vi "MeasureDC120629.vi"() -> ()   [LabVIEW 2011]
uses:
  Sub VIs/Trap cluster.ctl
  <vilib>/Utility/inputDevices.llb/closeKeyboard.vi
  <vilib>/Utility/inputDevices.llb/keyboardAcquire.vi
  <vilib>/Utility/file.llb/Write To Spreadsheet File (DBL).vi
  <vilib>/vision/driver/NI_Vision_Acquisition_Software.lvlib
panel:
  in  "Generate hologram":bool
  in  "ok 2":bool caption="Mark the center of \nthe spot using the \nzoom and the point\ntool, then click this \nbutton"
  in  "Run calibration 2":bool
  in  "e_desired":sgl=0.5
  in  "View Licence":bool
  in  "Stop program":bool
  out "Camera enabled":bool
  out "SLM enabled":bool
  in  "Hologram generation":cluster{"Method":i32, "Iterations":i32}={"Method"=0, "Iterations"=10} {"Method" items=["Lenses & Gratings (3D)", " Gerchberg-Saxton (3D)", "Gerchberg-Saxton FFT (2D)"]}
  in  "Display hologram\nand computed \nimage plane":bool=TRUE
  in  "ROI":T1={"Global Rectangle"=[568, 568, 719, 569], "Contours"=[{"Contour Type"=0, "ROI Type"=1, "Points"=[568, 568]}, {"Contour Type"=0, "ROI Type"=1, "Points"=[642, 568]}, {"Contour Type"=0, "ROI Type"=1, "Points"=[718, 568]}]}
  out "Image":T2(plugin-control)
  in  "Spots x":i32
  in  "Spots y":i32
  in  "Cancel calibration 2":bool
  in  "separation step":i32=1 min=1
  in  "max separation":i32=40
  in  "min separation":i32=30
  in  "Measure":bool
  in  "#images":i32=1
  out "Step number":i32
  in  "Move one spot":bool
  in  "y":dbl=100.0 min=1e-22
  in  "Filename":string="test"
  out "appended path":path=path "C:/Users/Martin/Dropbox/GU/CUDA/GenerateHologramCUDA/LabVIEW/MartinDC/Measurements/test0_0.bmp"
  in  "File Path":path=path "C:/Users/Martin/Dropbox/GU/CUDA/GenerateHologramCUDA/LabVIEW/MartinDC/Measurements"
  in  "Show image":bool=TRUE
  in  "ROI size":dbl=2.0 min=2.0 step=2.0
  out "Calculated image plane":dbl[][](graph)
  out "Current trap pos":T3={"X (IMAQ)"=[555.0, 642.5, 730.0, 555.0, 642.5, 730.0, 555.0, 642.5, 730.0], "Y (IMAQ)"=[555.0, 555.0, 555.0, 642.5, 642.5, 642.5, 730.0, 730.0, 730.0], "Z"=[0.0, 0.0, 0.0, 0.0, 0.0, 0.0, 0.0, 0.0, 0.0], "Amplitudes"=[1.0, 1.0, 1.0, 1.0, 1.0, 1.0, 1.0, 1.0, 1.0], "Trap number"=[0, 1, 2, 3, 4, 5, 6, 7, 8], "ROI number"=[0, 1, 2, 3, 4, 5, 6, 7, 8], "Number of traps"=9, "Group"=[FALSE, FALSE, FALSE, FALSE, FALSE, FALSE, FALSE, FALSE, FALSE]}
  out "NI Vision error":errorcluster
  out "CUDA/SLM error":errorcluster
  in  "Display path":bool=TRUE
  out "Displayed Hologram":u8[][](graph)
  in  "Coordinate mapping \n(IMAQ to SLM)":T4={"sX"=-256.0, "sY"=-256.0, "sZ"=0.0, "cX"=0.4, "cY"=0.4, "cZ"=1.0}
  in  "Switch X/Y":bool
  # "Martin\nPersson 2011"
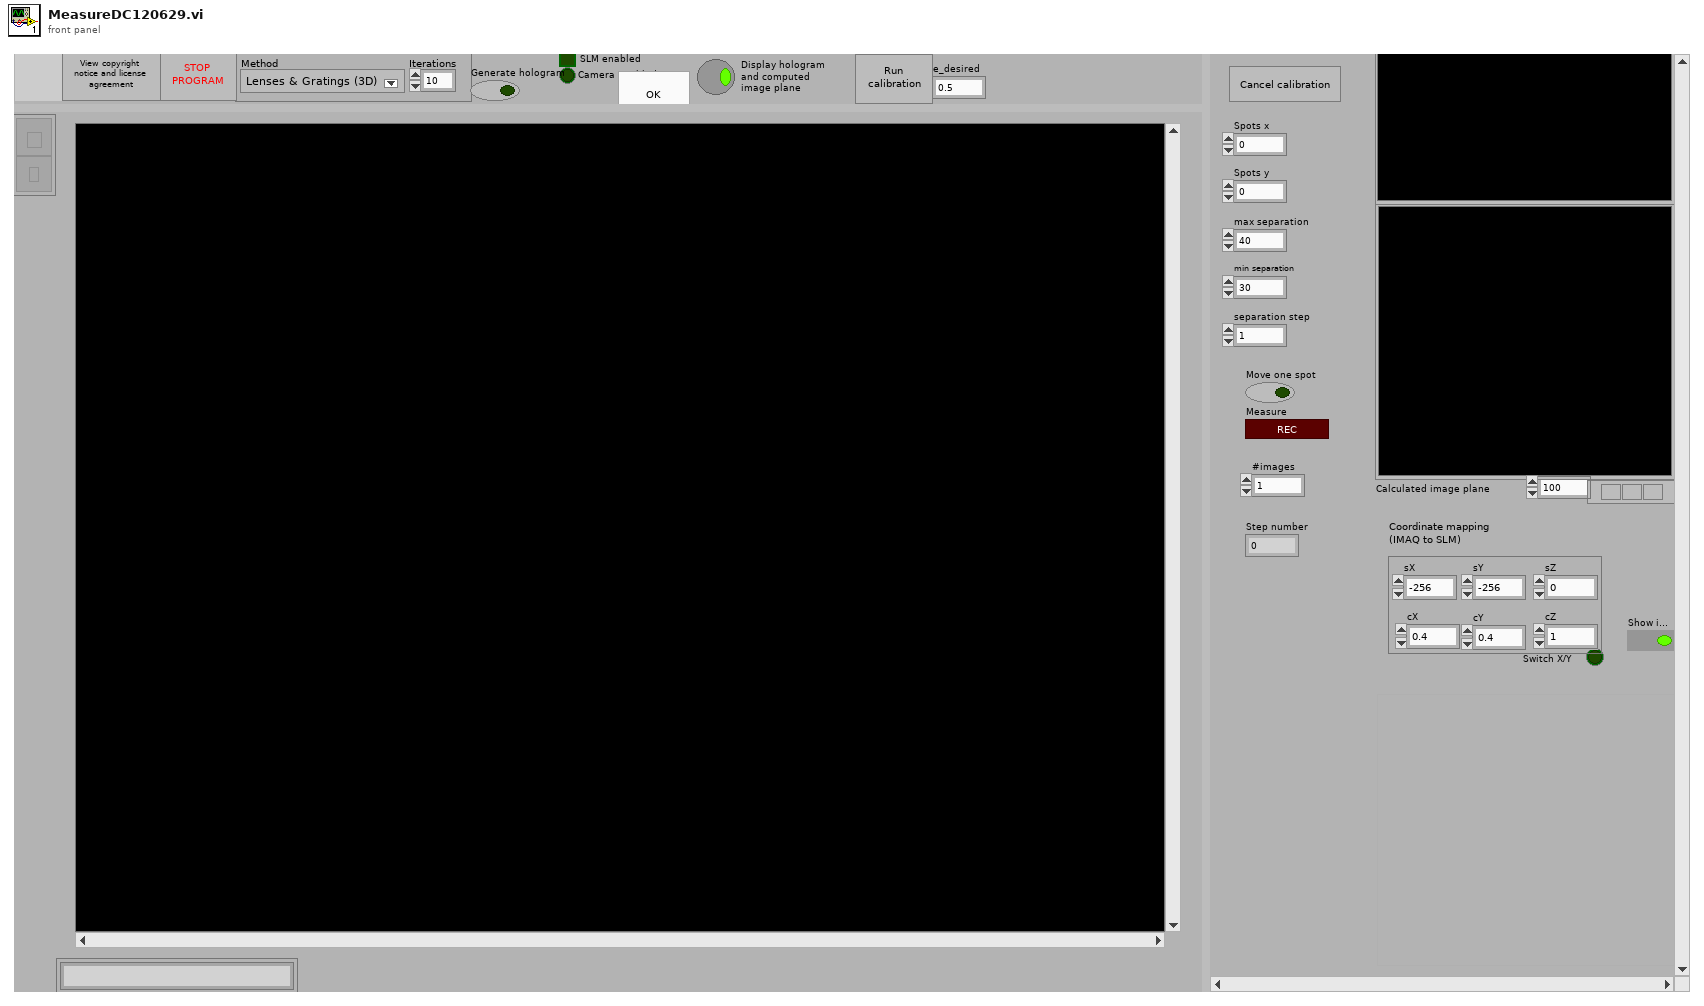
[diagram p1: front panel]
types:
  T1 = cluster{"Global Rectangle":i32[], "Contours":cluster{"Contour Type":u32, "ROI Type":u32, "Points":i32[]}[]}
  T2 = typedef "IMAQ Image.ctl" = refnum<image>
  T3 = typedef "Trap cluster.ctl" = cluster{"X (IMAQ)":dbl[], "Y (IMAQ)":dbl[], "Z":dbl[], "Amplitudes":dbl[], "Trap number":i32[], "ROI number":i32[], "Number of traps":i32, "Group":bool[]}
  T4 = cluster{"sX":dbl, "sY":dbl, "sZ":dbl, "cX":dbl, "cY":dbl, "cZ":dbl}
  T5 = cluster{"Centroid X":dbl[], "Centroid Y":dbl[], "Acquired Buffer Number":u32}
  T6 = typedef "IMAQdx.ctl" = refnum<k21>
  T7 = enum16{"0", "1", "2", "3", "4", "5", "6", "7", "8", "9", "A", "B", "C", "D", "E", "F", "G", "H", "I", "J", "K", "L", "M", "N", "O", "P", "Q", "R", "S", "T", "U", "V", "W", "X", "Y", "Z", "F1", "F2", "F3", "F4", "F5", "F6", "F7", "F8", "F9", "F10", "F11", "F12", "F13", "F14", "F15", "ADD", "BACK", "BACKSLASH", "CAPITAL", "COMMA", "DECIMAL", "DELETE", "DIVIDE", "DOWN", "END", "EQUALS", "ESCAPE", "GRAVE (`)", "HOME", "INSERT", "LBRACKET", "LCONTROL", "LEFT", "L ALT", "LSHIFT", "LWIN", "MINUS", "MULTIPLY", "NEXT", "NUMLOCK", "NUMPAD_0", "NUMPAD_1", "NUMPAD_2", "NUMPAD_3", "NUMPAD_4", "NUMPAD_5", "NUMPAD_6", "NUMPAD_7", "NUMPAD_8", "NUMPAD_9", "PAUSE", "PERIOD", "PRIOR (PG UP)", "RBRACKET", "RCONTROL", "RETURN", "RIGHT", "R ALT", "RSHIFT", "RWIN", "SCROLL", "SEMICOLON", "SLASH", "SPACE", "SUBTRACT", "TAB", "UP", "ENTER (num pad)", "' (quote)"}[]
  T8 = typedef "LVRectTypeDef.ctl" = cluster{"left":i16, "top":i16, "right":i16, "bottom":i16}
  T9 = cluster{"Contour Type":u32, "ROI Type":u32, "Points":i32[]}[]
  T10 = cluster{"Contour Type":u32, "ROI Type":u32, "Points":i32[]}
  T11 = typedef "Semaphore RefNum" = refnum<k1>
  T12 = typedef "Image Type" = u32
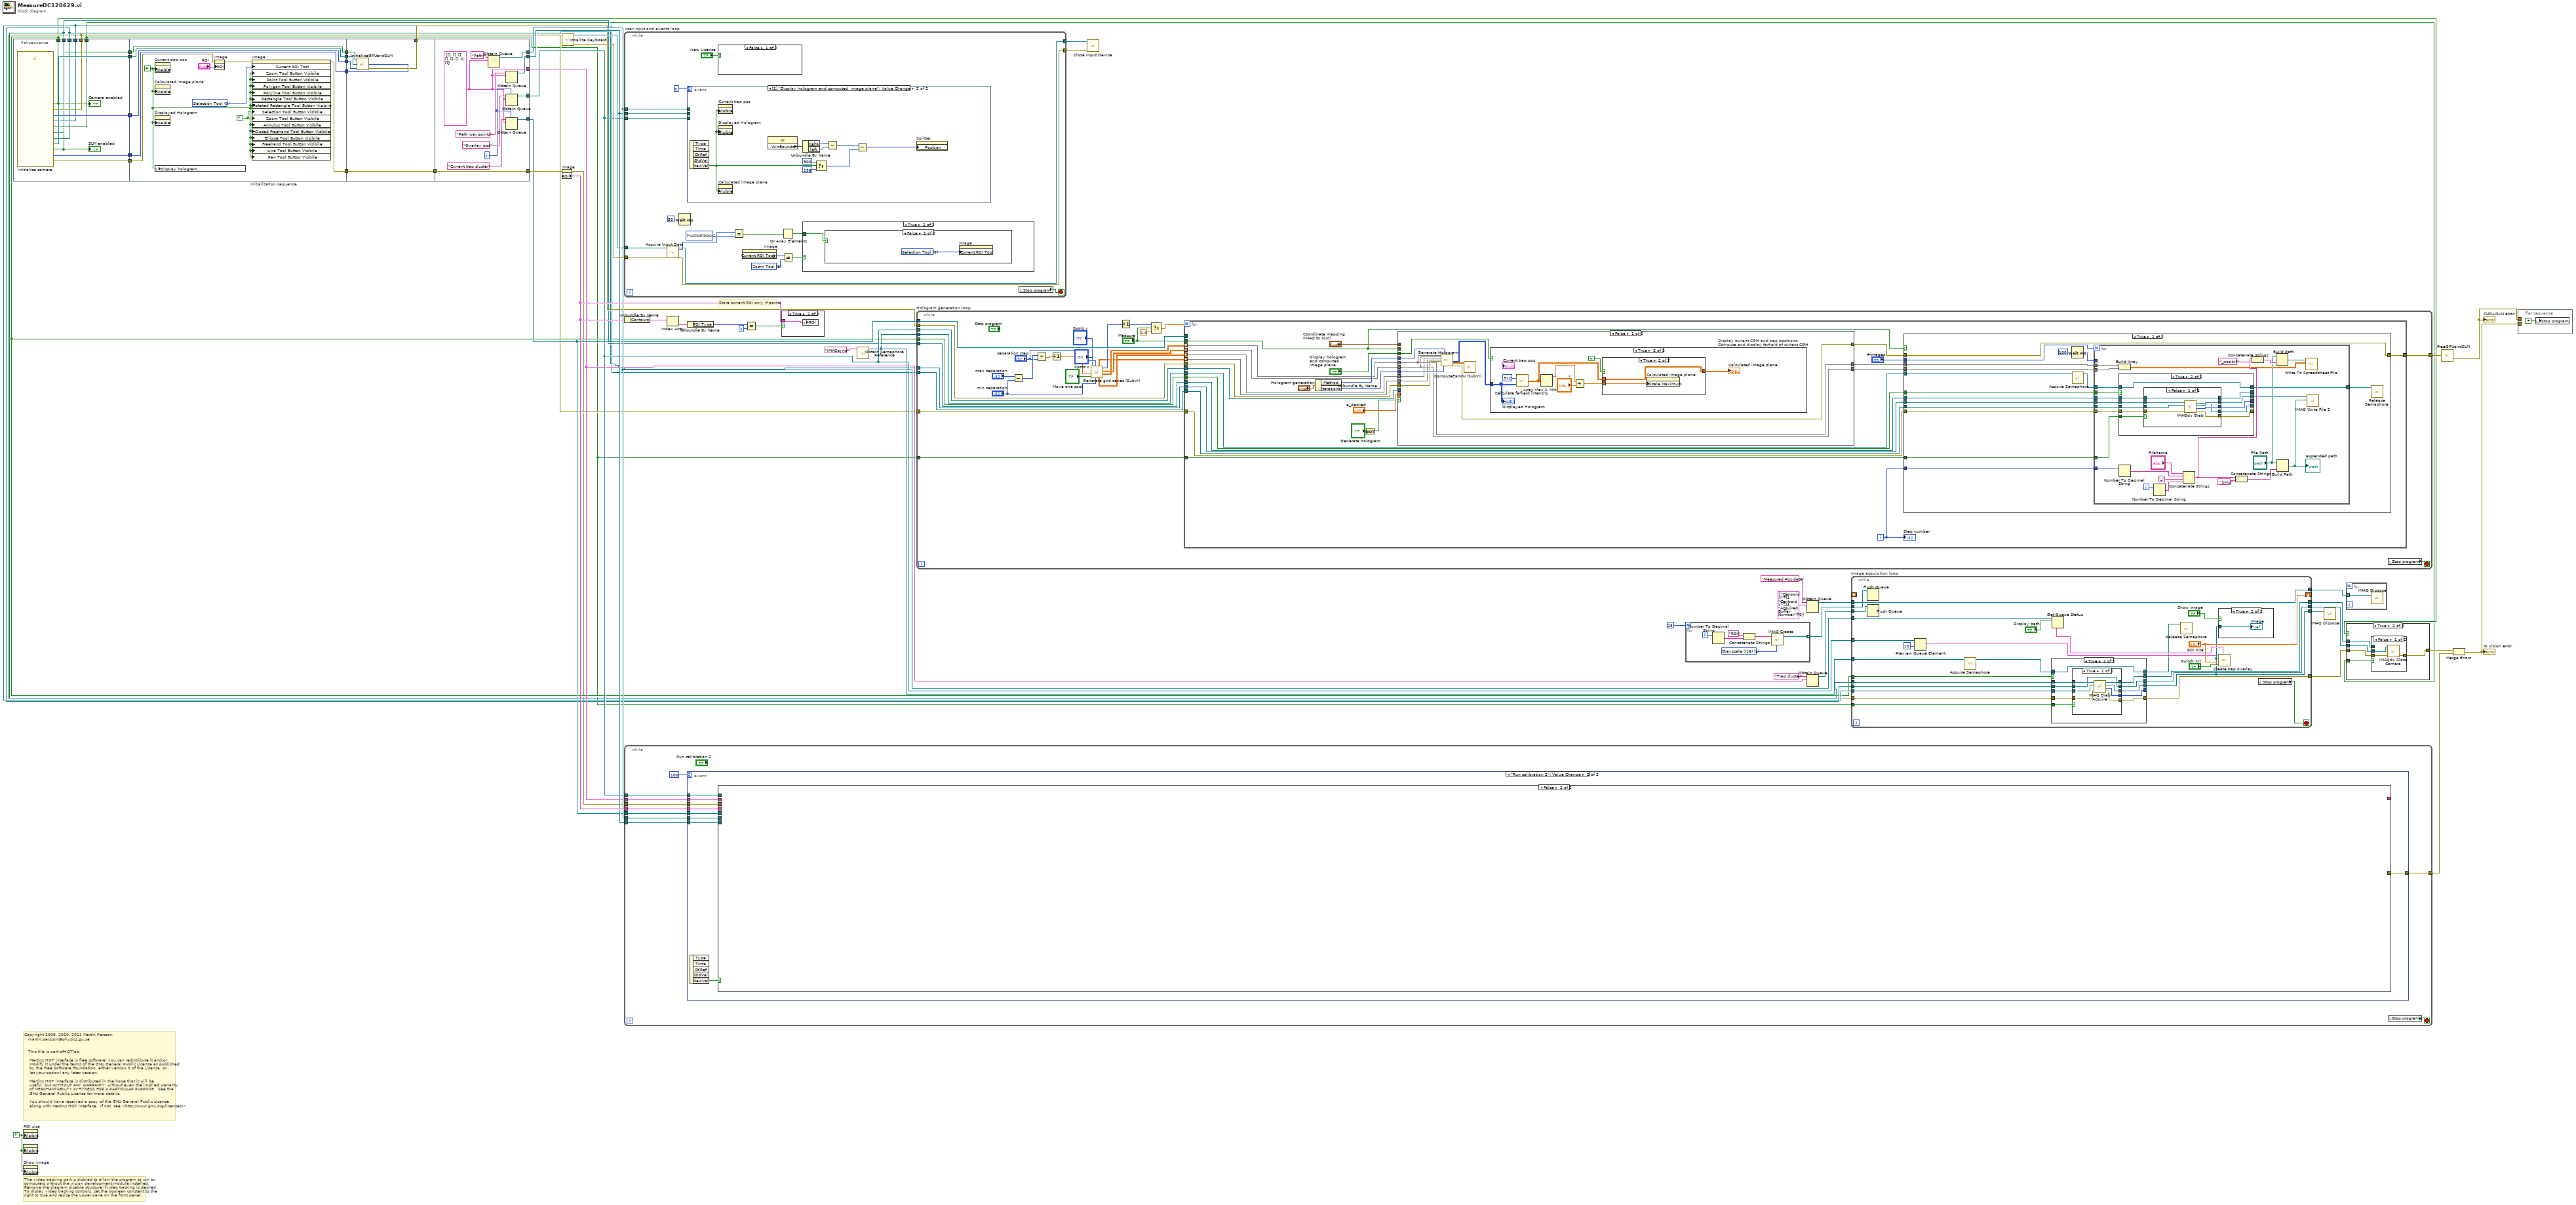
[diagram p0: block diagram]
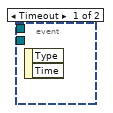
[diagram p2: hidden frame]
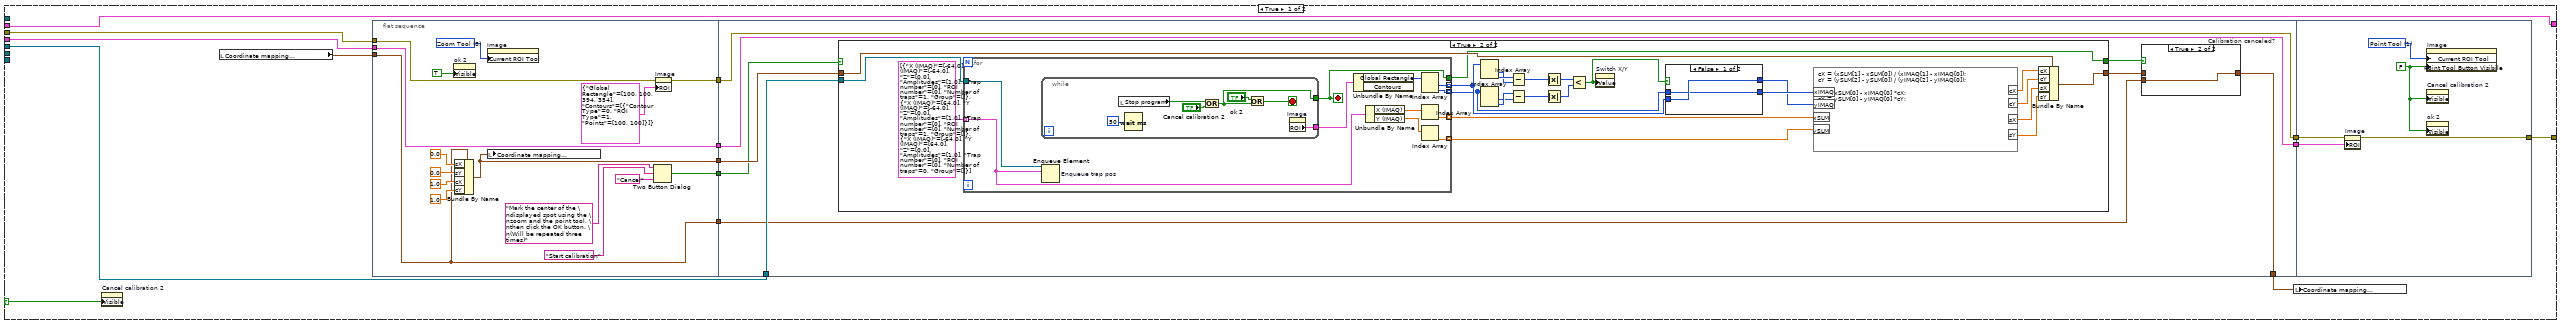
[diagram p3: hidden frame]
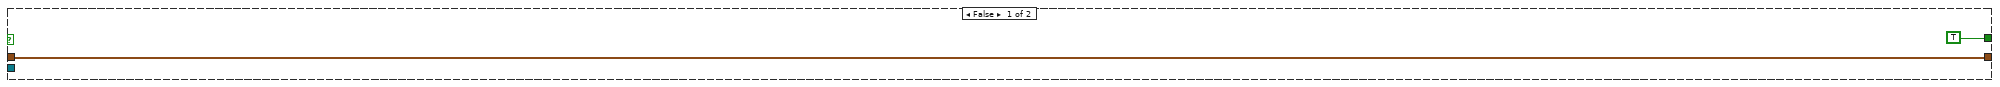
[diagram p5: hidden frame]
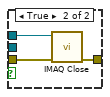
[diagram p8: hidden frame]
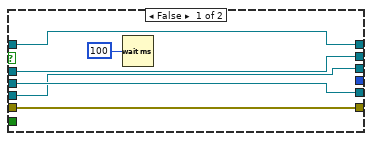
[diagram p10: hidden frame]
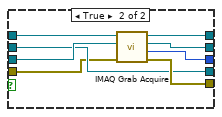
[diagram p11: hidden frame]
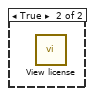
[diagram p15: hidden frame]
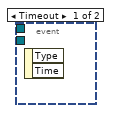
[diagram p16: hidden frame]
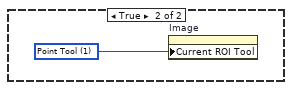
[diagram p18: hidden frame]
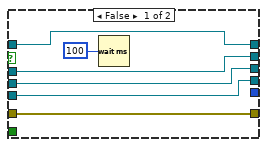
[diagram p20: hidden frame]
diagram:
  w42 = TRUE ("Visible")
  # "Copyright 2009, 2010, 2011 Martin Persson \n   martin.persson@physics.gu.se\n\n\n   This file is part ofHOTlab.\n\n    Martins HOT interface is free software: you can redistribute it and/or \n    modify it under the terms of the GNU General Public License as published \n    by the Free Software Foundation, either version 3 of the License, or\n    (at your option) any later version.\n\n    Martins HOT interface is distributed in the hope that it will be \n    useful, but WITHOUT ANY WARRANTY; without even the implied warranty\n    of MERCHANTABILITY or FITNESS FOR A PARTICULAR PURPOSE.  See the\n    GNU General Public License for more details.\n\n    You should have received a copy of the GNU General Public License\n    along with Martins HOT interface.  If not, see <http://www.gnu.org/licenses/>."
  # "Store current ROI only if points"
  # "The video tracking part is disbled to allow the program to run on\ncomputers without the vision development module installed. \nRemove the diagram disable structure ifvideo tracking is desired. \nTo diplay video tracking controls, set the boolean constant to the \nright to true And resize the upper pane on the front panel."
  n1 = flat-sequence "Initialization sequence" {
    tunnel: [w57] -> w27
    tunnel: [w66] -> w26
    tunnel: [w65] -> w25
    tunnel: [w64] -> w24
    tunnel: [w63] -> w23
    tunnel: [w62] -> w7
    tunnel: [w61] -> w8
    tunnel: [w60] -> w6
    tunnel: [w59] -> w4
    tunnel: [w58] -> w9
    tunnel: [w56] -> w5
    tunnel: w27 -> [w74]
    tunnel: w26 -> [w72]
    tunnel: w25 -> [w77]
    tunnel: w24 -> [w76]
    tunnel: w23 -> [w75]
    tunnel: [w74] -> w16
    tunnel: [w67] -> w15
    tunnel: [w77] -> w13
    tunnel: [w76] -> w12
    tunnel: [w75] -> w11
    tunnel: w16 -> [w80]
    tunnel: w15 -> [w83]
    tunnel: [w83] -> w14
    tunnel: w13 -> [w81]
    tunnel: w12 -> [w82]
    tunnel: w11 -> [w79]
    tunnel: [w78] -> w10
    tunnel: [w94] -> w22
    tunnel: w14 -> [w94]
    tunnel: [w92] -> w21
    tunnel: [w90] -> w20
    tunnel: [w88] -> w19
    tunnel: [w87] -> w18
    tunnel: [w84] -> w17
    frame #0 {
      n2 = call "Initialize camera.vi"() -> ("CUDA device ID"=w64:i32, "IMAQdx Session Out"=w61:T6, "TrueFrame out"=w65:i32, "IMAQ camera"=w59:bool, "Image reference out"=w62:T2, "SLM enabled"=w57:bool, "Camera enabled"=w56:bool, "Vision error out"=w66:errorcluster, "LUT path out"=w63:path, "IMAQ Session Out"=w58:refnum<k11>, "Camera error"=w60:errorcluster)  [unwired: 5 in]
      "Camera enabled" <- w56
      "SLM enabled" <- w57
    }
    frame #1 {
      w70 = TRUE ("ROI Tool Buttons Visibile:Zoom Tool Button Visible")
      w71 = FALSE ("ROI Tool Buttons Visibile:Zoom Tool Button Visible")
      w69 = u32 0 items=["Zoom Tool"=8, "Selection Tool"=0, "Pan Tool"=9, "Point Tool"=1, "Line Tool"=2, "Rectangle Tool"=3, "Rotated Rectangle Tool"=12, "Polyline Tool"=10, "Polygon Tool"=5, "Freehand Tool"=11, "Closed Freehand Tool"=6, "Ellipse Tool"=4, "Annulus Tool"=7] ("Current ROI Tool")
      n3 = property on="Current trap pos" class="Clust (strict)"("Visible"=w71) -> ()  [unwired: 2 in, 2 out]
      n4 = property on="Calculated image plane" class="IntGraph (strict)"("Visible"=w71) -> ()  [unwired: 2 in, 2 out]
      n5 = property on="Displayed Hologram" class="IntGraph (strict)"("Visible"=w71) -> ()  [unwired: 2 in, 2 out]
      n6 = local write "Display hologram\nand computed \nimage plane"(w71) -> ()
      n7 = property on="Image" class="ImageControl"(error in=w72, "ROI"="ROI") -> (error out=w68:errorcluster)  [unwired: 1 in, 1 out]
      n8 = property on="Image" class="ImageControl"(error in=w68, "Current ROI Tool"=w69, "Zoom Tool Button Visibile"=w71, "Point Tool Button Visibile"=w71, "Polygon Tool Button Visibile"=w71, "Polyline Tool Button Visibile"=w71, "Rectangle Tool Button Visibile"=w71, "Rotated Rectangle Tool Button Visibile"=w71, "Selection Tool Button Visibile"=w70, "Zoom Tool Button Visibile"=w70, "Annulus Tool Button Visibile"=w71, "Closed Freehand Tool Button Visibile"=w71, "Ellipse Tool Button Visibile"=w71, "Freehand Tool Button Visibile"=w71, "Line Tool Button Visibile"=w71, "Pan Tool Button Visibile"=w71) -> (error out=w67:errorcluster)  [unwired: 1 in, 1 out]
    }
    frame #2 {
      n9 = call "InitializeGPUandSLM.vi"("TrueFrame"=w81, "deviceId"=w82, "Path to LUT file"=w79, "SLM enabled"=w80) -> ("CUDA/SLM error"=w78:errorcluster)  [unwired: 1 out]
    }
    frame #3 {
      w85 = 1 ("max queue size (-1, unlimited)")
      w84 = T3 {"X (IMAQ)"=[], "Y (IMAQ)"=[], "Z"=[], "Amplitudes"=[], "Trap number"=[], "ROI number"=[], "Number of traps"=0, "Group"=[]} ("output cluster 2")
      n10 = Obtain Queue(name (unnamed)="Path", element data type=w84) -> (queue out=w92:refnum<queue>)  [unwired: 3 in, 2 out]
      n11 = Obtain Queue(name (unnamed)="Path waypoints", element data type=w84) -> (queue out=w90:refnum<queue>)  [unwired: 3 in, 2 out]
      n12 = Obtain Queue(max queue size (-1, unlimited)=w85, name (unnamed)="Overlay pos", element data type=w84) -> (queue out=w87:refnum<queue>)  [unwired: 2 in, 2 out]
      n13 = Obtain Queue(max queue size (-1, unlimited)=w85, name (unnamed)="Current trap cluster", element data type=w84) -> (queue out=w88:refnum<queue>)  [unwired: 2 in, 2 out]
    }
  }
  n14 = property on="ROI size" class="DigNum (strict)"("Visible"=w42) -> ()  [unwired: 2 in, 2 out]
  n15 = property on="Measure" class="Bool"("Visible"=w42) -> ()  [unwired: 2 in, 2 out]
  n16 = property on="Show image" class="Bool (strict)"("Visible"=w42) -> ()  [unwired: 2 in, 2 out]
  n17 = call <vilib>:"Intialize Keyboard.vi"() -> ("error out"=w29:errorcluster, "device ID"=w55:refnum<k1>)  [unwired: 1 in, 9 out]
  n18 = property on="Image" class="ImageControl"(error in=w22) -> (error out=w1:errorcluster, "ROI"=w36:T1)  [unwired: 1 in, 1 out]
  n19 = while "User input and events loop" {
    tunnel: w55 -> [w112]
    tunnel: w18 -> [w101]
    tunnel: w20 -> [w100]
    tunnel: w21 -> [w99]
    tunnel: [w98] -> w30
    tunnel: w29 -> [w97]
    tunnel: [w96] -> w28
    stop <- w104 stop-if-true
    w109 = u32 8 items=["Zoom Tool"=8, "Selection Tool"=0, "Pan Tool"=9, "Point Tool"=1, "Line Tool"=2, "Rectangle Tool"=3, "Rotated Rectangle Tool"=12, "Polyline Tool"=10, "Polygon Tool"=5, "Freehand Tool"=11, "Closed Freehand Tool"=6, "Ellipse Tool"=4, "Annulus Tool"=7] ("Current ROI Tool")
    w106 = T7 [enum."LCONTROL"] items=["0", "1", "2", "3", "4", "5", "6", "7", "8", "9", "A", "B", "C", "D", "E", "F", "G", "H", "I", "J", "K", "L", "M", "N", "O", "P", "Q", "R", "S", "T", "U", "V", "W", "X", "Y", "Z", "F1", "F2", "F3", "F4", "F5", "F6", "F7", "F8", "F9", "F10", "F11", "F12", "F13", "F14", "F15", "ADD", "BACK", "BACKSLASH", "CAPITAL", "COMMA", "DECIMAL", "DELETE", "DIVIDE", "DOWN", "END", "EQUALS", "ESCAPE", "GRAVE (`)", "HOME", "INSERT", "LBRACKET", "LCONTROL", "LEFT", "L ALT", "LSHIFT", "LWIN", "MINUS", "MULTIPLY", "NEXT", "NUMLOCK", "NUMPAD_0", "NUMPAD_1", "NUMPAD_2", "NUMPAD_3", "NUMPAD_4", "NUMPAD_5", "NUMPAD_6", "NUMPAD_7", "NUMPAD_8", "NUMPAD_9", "PAUSE", "PERIOD", "PRIOR (PG UP)", "RBRACKET", "RCONTROL", "RETURN", "RIGHT", "R ALT", "RSHIFT", "RWIN", "SCROLL", "SEMICOLON", "SLASH", "SPACE", "SUBTRACT", "TAB", "UP", "ENTER (num pad)", "' (quote)"] ("keys pressed")
    n20 = call-poly <vilib>:"Acquire Input Data.vi"("device ID"=w112, "error in (no error)"=w97) -> ("device ID"=w98:refnum<k1>, "keys pressed"=w105:T7, "error out"=w96:errorcluster)  [unwired: 15 out]
    n21 = Wait (ms)(milliseconds to wait=u32 50) -> ()  [unwired: 1 out]
    n22 = event shown="[1] \"Display hologram\nand computed \nimage plane\": Value Change" {
      selector: _ -> [_ _]
      dyn-events: _ -> [_ _]
      timeout: 0 -> [_ _]
      tunnel: w101 -> [_ _]
      tunnel: w100 -> [_ _]
      tunnel: w99 -> [_ _]
      event Timeout {
        n23 = event-data() -> ()  [unwired: 1 in, 2 out]
      }
      event "Display hologram\nand computed \nimage plane": Value Change {
        n24 = event-data() -> ("NewVal"=w114:bool)  [unwired: 1 in, 4 out]
        n25 = property on="Current trap pos" class="Clust (strict)"("Visible"=w114) -> ()  [unwired: 2 in, 2 out]
        n26 = property on="Displayed Hologram" class="IntGraph (strict)"("Visible"=w114) -> ()  [unwired: 2 in, 2 out]
        n27 = property on="Calculated image plane" class="IntGraph (strict)"("Visible"=w114) -> ()  [unwired: 2 in, 2 out]
        n28 = property on="Property Node" class="VI"() -> ("Front Panel.WinBounds"=w121:T8)  [unwired: 2 in, 2 out]
        n29 = Unbundle By Name(w121) -> ("right"=w120:i16, "left"=w119:i16)
        n30 = Select(t=i16 500 ("x-y"), s=w114, f=i16 196 ("x-y")) -> (s? t:f=w113:i16)
        n31 = Subtract(x=w120, y=w119) -> (x-y=w118:i16)
        n32 = Subtract(x=w118, y=w113) -> (x-y=w117:i16)
        n33 = property on="Splitter" class="Splitter"("Position"=w117) -> ()  [unwired: 2 in, 2 out]
      }
    }
    n34 = case shown="False" "View Licence" {
      frame False {
      }
      frame True {
        n35 = call "View license.vi"() -> ()  [unwired: 1 in]
      }
    }
    n36 = Equal?(x=w105, y=w106) -> (x = y?=w107:bool[])
    n37 = property on="Image" class="ImageControl"() -> ("Current ROI Tool"=w108:u32)  [unwired: 2 in, 2 out]
    n38 = Or Array Elements(Boolean array=w107) -> (logical OR=w111:bool)
    n39 = Not Equal?(x=w108, y=w109) -> (x != y?=w110:bool)
    n40 = case shown="True" w110 {
      tunnel: w111 -> [_ w122]
      frame False {
      }
      frame True {
        n41 = case shown="False" w122 {
          frame False {
            w123 = u32 0 items=["Zoom Tool"=8, "Selection Tool"=0, "Pan Tool"=9, "Point Tool"=1, "Line Tool"=2, "Rectangle Tool"=3, "Rotated Rectangle Tool"=12, "Polyline Tool"=10, "Polygon Tool"=5, "Freehand Tool"=11, "Closed Freehand Tool"=6, "Ellipse Tool"=4, "Annulus Tool"=7] ("Current ROI Tool")
            n42 = property on="Image" class="ImageControl"("Current ROI Tool"=w123) -> ()  [unwired: 2 in, 2 out]
          }
          frame True {
            w124 = u32 1 items=["Zoom Tool"=8, "Selection Tool"=0, "Pan Tool"=9, "Point Tool"=1, "Line Tool"=2, "Rectangle Tool"=3, "Rotated Rectangle Tool"=12, "Polyline Tool"=10, "Polygon Tool"=5, "Freehand Tool"=11, "Closed Freehand Tool"=6, "Ellipse Tool"=4, "Annulus Tool"=7] ("Current ROI Tool")
            n43 = property on="Image" class="ImageControl"("Current ROI Tool"=w124) -> ()  [unwired: 2 in, 2 out]
          }
        }
      }
    }
    n44 = local read "Stop program"() -> (w104:bool)
  }
  n45 = Unbundle By Name(w36) -> ("Contours"=w41:T9)
  n46 = while {
    tunnel: w36 -> [w134]
    tunnel: [w133] -> w34
    tunnel: w21 -> [w132]
    tunnel: w20 -> [w131]
    tunnel: w19 -> [w130]
    tunnel: w18 -> [w129]
    tunnel: w17 -> [w128]
    tunnel: w1 -> [w127]
    stop <- w125 stop-if-true
    n47 = event shown="[1] \"Run calibration 2\": Value Change" {
      selector: _ -> [_ _]
      dyn-events: _ -> [_ _]
      timeout: 100 -> [_ _]
      tunnel: w134 -> [_ w143]
      tunnel: [_ w142] -> w133
      tunnel: w132 -> [_ w141]
      tunnel: w131 -> [_ w140]
      tunnel: w130 -> [_ w139]
      tunnel: w129 -> [_ w138]
      tunnel: w128 -> [_ w137]
      tunnel: w127 -> [_ w136]
      event Timeout {
        n48 = event-data() -> ()  [unwired: 1 in, 2 out]
      }
      event "Run calibration 2": Value Change {
        n49 = event-data() -> ("NewVal"=w135:bool)  [unwired: 1 in, 4 out]
        n50 = case shown="False" w135 {
          selector: w135 -> [w145 _]
          tunnel: w140 -> [_ _]
          tunnel: w137 -> [w144 _]
          tunnel: [w144 _] -> _
          tunnel: w139 -> [w154 _]
          tunnel: w141 -> [_ _]
          tunnel: w138 -> [_ _]
          tunnel: w143 -> [w153 _]
          tunnel: w136 -> [w149 _]
          tunnel: [w146 _] -> w142
          frame True {
            n51 = property on="Cancel calibration 2" class="Bool"("Visible"=w145) -> ()  [unwired: 2 in, 2 out]
            n52 = local read "Coordinate mapping \n(IMAQ to SLM)"() -> (w152:T4)
            n53 = flat-sequence {
              tunnel: [w168] -> w158
              tunnel: [w170] -> w157
              tunnel: w153 -> [w168]
              tunnel: w152 -> [w162]
              tunnel: [w159] -> w151
              tunnel: [w162] -> w150
              tunnel: w149 -> [w161]
              tunnel: [w160] -> w147
              tunnel: [w183] -> w156
              tunnel: w158 -> [w183]
              tunnel: w157 -> [w177]
              tunnel: [w179] -> w155
              tunnel: w154 -> [w182]
              tunnel: w151 -> [w181]
              tunnel: w150 -> [w178]
              tunnel: [w175] -> w148
              tunnel: w147 -> [w175]
              tunnel: w156 -> [w238]
              tunnel: w148 -> [w236]
              tunnel: [w235] -> w146
              frame #0 {
                w171 = u32 8 items=["Zoom Tool"=8, "Selection Tool"=0, "Pan Tool"=9, "Point Tool"=1, "Line Tool"=2, "Rectangle Tool"=3, "Rotated Rectangle Tool"=12, "Polyline Tool"=10, "Polygon Tool"=5, "Freehand Tool"=11, "Closed Freehand Tool"=6, "Ellipse Tool"=4, "Annulus Tool"=7] ("Current ROI Tool")
                n54 = property on="ok 2" class="Bool"("Visible"=TRUE ("ROI Tool Buttons Visibile:Zoom Tool Button Visible")) -> ()  [unwired: 2 in, 2 out]
                n55 = Bundle By Name(cluster=w162, "sX"=0.0, "sY"=0.0, "cX"=1.0 ("sX"), "cY"=1.0) -> (w159:T4)
                n56 = property on="Image" class="ImageControl"("Current ROI Tool"=w171) -> ()  [unwired: 2 in, 2 out]
                n57 = local write "Coordinate mapping \n(IMAQ to SLM)"(w159) -> ()
                n58 = Two Button Dialog(message="Mark the center of the \ndisplayed spot using the \nzoom and the point tool, \nthen click the OK button. \n(Will be repeated three times)", 1:"Cancel" ("F button name (\"Cancel\")"), 2:"Start calibration" ("T button name (\"OK\")")) -> (T button?=w170:bool)
                n59 = property on="Image" class="ImageControl"(error in=w161, "ROI"=T1 {"Global Rectangle"=[100, 100, 394, 354], "Contours"=[{"Contour Type"=0, "ROI Type"=1, "Points"=[100, 100]}]} ("ROI 2")) -> (error out=w160:errorcluster)  [unwired: 1 in, 1 out]
              }
              frame #1 {
                n60 = case shown="True" w177 {
                  tunnel: w181 -> [w187 w198]
                  tunnel: [w187 w193] -> w180
                  tunnel: w182 -> [_ w189]
                  tunnel: [TRUE ("Stop program") w188] -> w176
                  frame False {
                  }
                  frame True {
                    n61 = for {
                      tunnel: [w225] -> w207 mode=indexing
                      tunnel: [w224] -> w206 mode=indexing
                      tunnel: T3[] [{"X (IMAQ)"=[-64.0], "Y (IMAQ)"=[-64.0], "Z"=[0.0], "Amplitudes"=[1.0], "Trap number"=[0], "ROI number"=[0], "Number of traps"=1, "Group"=[]}, {"X (IMAQ)"=[64.0], "Y (IMAQ)"=[-64.0], "Z"=[0.0], "Amplitudes"=[1.0], "Trap number"=[0], "ROI number"=[0], "Number of traps"=1, "Group"=[]}, {"X (IMAQ)"=[-64.0], "Y (IMAQ)"=[64.0], "Z"=[0.0], "Amplitudes"=[1.0], "Trap number"=[0], "ROI number"=[0], "Number of traps"=0, "Group"=[]}] -> [w222] mode=indexing
                      tunnel: [w219] -> w191 mode=indexing
                      tunnel: [w217] -> w190 mode=indexing
                      tunnel: w189 -> [w221]
                      tunnel: [w216] -> w188
                      stop <- w216 stop-if-true
                      n62 = while {
                        tunnel: [w232] -> w223
                        tunnel: [w228] -> w216
                        stop <- w230 stop-if-true
                        n63 = local read "Stop program"() -> (w229:bool)
                        n64 = Wait (ms)(milliseconds to wait=u32 50) -> ()  [unwired: 1 out]
                        n65 = Or(x=w229, y="Cancel calibration 2") -> (x .or. y?=w228:bool)
                        n66 = Or(x="ok 2", y=w228) -> (x .or. y?=w230:bool)
                        n67 = property on="Image" class="ImageControl"() -> ("ROI"=w232:T1)  [unwired: 2 in, 2 out]
                      }
                      n68 = Enqueue Element "Enqueue trap pos"(queue=w221, element=w222) -> ()  [unwired: 2 in, 3 out]
                      n69 = Unbundle By Name(w223) -> ("Global Rectangle"=w226:i32[])  [unwired: 1 out]
                      n70 = Unbundle By Name(w222) -> ("X (IMAQ)"=w220:dbl[], "Y (IMAQ)"=w218:dbl[])
                      n71 = Index Array(array=w226) -> (element #1=w225:i32, element #2=w224:i32)  [unwired: 2 in]
                      n72 = Index Array(array=w220) -> (element=w219:dbl)  [unwired: 1 in]
                      n73 = Index Array(array=w218) -> (element=w217:dbl)  [unwired: 1 in]
                    }
                    n74 = Index Array(array=w207) -> (element #1=w210:i32, element #2=w211:i32)  [unwired: 2 in]
                    n75 = Index Array(array=w206) -> (element #1=w208:i32, element #2=w209:i32)  [unwired: 2 in]
                    n76 = Subtract(x=w211, y=w210) -> (x-y=w203:i32)
                    n77 = Subtract(x=w209, y=w208) -> (x-y=w201:i32)
                    n78 = Absolute Value(x=w203) -> (abs(x)=w202:i32)
                    n79 = Absolute Value(x=w201) -> (abs(x)=w200:i32)
                    n80 = Less?(x=w202, y=w200) -> (x < y?=w199:bool)
                    n81 = property on="Switch X/Y" class="Bool (strict)"("Value"=w199) -> ()  [unwired: 2 in, 2 out]
                    n82 = case shown="False" w199 {
                      tunnel: w207 -> [w213 w215]
                      tunnel: w206 -> [w212 w214]
                      tunnel: [w212 w215] -> w204
                      tunnel: [w213 w214] -> w205
                      frame False {
                      }
                      frame True {
                      }
                    }
                    n83 = formula code="cX = (xSLM[1] - xSLM[0]) / (xIMAQ[1] - xIMAQ[0]); \ncY = (ySLM[2] - ySLM[0]) / (yIMAQ[2] - yIMAQ[0]); \n\nsX = xSLM[0] - xIMAQ[0] *cX;\nsY = ySLM[0] - yIMAQ[0] *cY;"("xIMAQ"=w205, "yIMAQ"=w204, "xSLM"=w191, "ySLM"=w190) -> ("cX"=w197:dbl, "cY"=w196:dbl, "sX"=w195:dbl, "sY"=w194:dbl)
                    n84 = Bundle By Name(cluster=w198, "cX"=w197, "cY"=w196, "sX"=w195, "sY"=w194) -> (w193:T4)
                  }
                }
                n85 = case "Calibration canceled?" shown="True" w176 {
                  tunnel: w180 -> [w184 _]
                  tunnel: [w184 w185] -> w179
                  tunnel: w178 -> [_ w185]
                  frame False {
                  }
                  frame True {
                  }
                }
              }
              frame #2 {
                w234 = FALSE ("ROI Tool Buttons Visibile:Zoom Tool Button Visible")
                w237 = u32 1 items=["Zoom Tool"=8, "Selection Tool"=0, "Pan Tool"=9, "Point Tool"=1, "Line Tool"=2, "Rectangle Tool"=3, "Rotated Rectangle Tool"=12, "Polyline Tool"=10, "Polygon Tool"=5, "Freehand Tool"=11, "Closed Freehand Tool"=6, "Ellipse Tool"=4, "Annulus Tool"=7] ("Current ROI Tool")
                n86 = property on="Image" class="ImageControl"(error in=w236, "ROI"=w238) -> (error out=w235:errorcluster)  [unwired: 1 in, 1 out]
                n87 = property on="Image" class="ImageControl"("Current ROI Tool"=w237, "Point Tool Button Visibile"=w234) -> ()  [unwired: 2 in, 2 out]
                n88 = property on="Cancel calibration 2" class="Bool"("Visible"=w234) -> ()  [unwired: 2 in, 2 out]
                n89 = property on="ok 2" class="Bool"("Visible"=w234) -> ()  [unwired: 2 in, 2 out]
              }
            }
            n90 = local write "Coordinate mapping \n(IMAQ to SLM)"(w155) -> ()
          }
          frame False {
          }
        }
      }
    }
    n91 = local read "Stop program"() -> (w125:bool)
  }
  n92 = Index Array(array=w41) -> (element=w40:T10)  [unwired: 1 in]
  n93 = Unbundle By Name(w40) -> ("ROI Type"=w39:u32)
  n94 = Equal?(x=w39, y=u32 1) -> (x = y?=w37:bool)
  n95 = case shown="True" w37 {
    tunnel: w36 -> [_ w239]
    frame False {
    }
    frame True {
      n96 = local write "ROI"(w239) -> ()
    }
  }
  n97 = call <vilib>:"Obtain Semaphore Reference.vi"("name (unnamed)"="IMAQsync") -> ("semaphore"=w2:T11)  [unwired: 4 in, 2 out]
  n98 = while "Hologram generation loop" {
    tunnel: w19 -> [w268]
    tunnel: w18 -> [w266]
    tunnel: w10 -> [w267]
    tunnel: [w261] -> w33
    tunnel: w9 -> [w265]
    tunnel: w8 -> [w264]
    tunnel: w7 -> [w263]
    tunnel: w6 -> [w262]
    tunnel: w5 -> [w260]
    tunnel: w4 -> [w259]
    tunnel: w2 -> [w258]
    stop <- w269 stop-if-true
    n99 = Subtract(x="max separation", y="min separation") -> (x-y=w253:i32)
    n100 = Divide(x=w253, y="separation step") -> (x/y=w252:dbl)
    n101 = Increment(x=w252) -> (x+1=w251:dbl)
    n102 = call "Generate grid series (SubVI).vi"("min separation"="min separation", "separation step"="separation step", "Move one spot"="Move one spot", "Number of steps"=w251, "Spots y"="Spots y", "Spots x"="Spots x") -> ("Y"=w246:sgl[][], "X"=w245:sgl[][], "Numeric out"=w248:i32, "Z"=w244:sgl[][], "I"=w243:sgl[][])  [unwired: 1 in]
    n103 = Increment(x=w248) -> (x+1=w247:i32)
    n104 = Select(t=w247, s="Measure", f=1.0) -> (s? t:f=w257:dbl)
    n105 = for {
      N: w257 -> [_]
      tunnel: w268 -> [_]
      tunnel: w267 -> [w292]
      tunnel: w266 -> [w290]
      tunnel: w265 -> [w288]
      tunnel: w264 -> [w287]
      tunnel: w263 -> [w286]
      tunnel: w262 -> [w285]
      tunnel: [w283] -> w261
      tunnel: w260 -> [w280]
      tunnel: w259 -> [w279]
      tunnel: w258 -> [w278]
      tunnel: "Measure" -> [w273]
      tunnel: w246 -> [w277] mode=indexing
      tunnel: w245 -> [w276] mode=indexing
      tunnel: w244 -> [w275] mode=indexing
      tunnel: w243 -> [w274] mode=indexing
      i -> [w272]
      n106 = Unbundle By Name("Hologram generation") -> ("Method"=w297:i32, "Iterations"=w296:i32)
      n107 = Not(x="Generate hologram") -> (.not. x?=w270:bool)
      n108 = case shown="False" w270 {
        tunnel: "Coordinate mapping \n(IMAQ to SLM)" -> [_ _]
        tunnel: "Display hologram\nand computed \nimage plane" -> [w381 _]
        tunnel: w297 -> [w383 _]
        tunnel: w296 -> [w382 _]
        tunnel: w290 -> [_ _]
        tunnel: w292 -> [w380 w395]
        tunnel: [w379 w395] -> w284
        tunnel: "e_desired" -> [_ _]
        tunnel: [w377 _] -> w282
        tunnel: [w376 _] -> w281
        tunnel: w277 -> [w377 _]
        tunnel: w276 -> [w376 _]
        tunnel: w275 -> [w375 _]
        tunnel: w274 -> [w374 _]
        tunnel: w273 -> [_ _]
        frame False {
          n109 = call "Generate Hologram.vi"("x"=w377, "y"=w376, "z"=w375, "spot_intensities"=w374, "CUDA/SLM error in"=w380, "N_iterations"=w382, "method"=w383) -> ("CGH out"=w384:u8[][], "weights"=w378:sgl[][], "CUDA/SLM error out"=w379:errorcluster)  [unwired: 17 in, 1 out]
          n110 = call "ComputeEandU (SubVI).vi"("weights in"=w378) -> ()  [unwired: 9 in, 2 out]
          n111 = case "Display current CGH and trap positions.\nCompute and display farfield of current CGH" shown="True" w381 {
            tunnel: w384 -> [_ w392]
            frame False {
            }
            frame True {
              n112 = call "Calculate farfield intensity.vi"("h_pSLM"=w392, "Numeric"=512) -> ("Calculated image plane"=w387:dbl[][])
              n113 = Array Max & Min(array=w387) -> (max value=w390:dbl)  [unwired: 3 out]
              n114 = Divide(x=w390, y="y") -> (x/y=w388:dbl)
              n115 = case shown="True" TRUE {
                tunnel: w388 -> [_ w394]
                tunnel: w387 -> [_ w393]
                tunnel: [_ w393] -> w386
                frame False {
                }
                frame True {
                  n116 = property on="Calculated image plane" class="IntGraph (strict)"("ZScale.Maximum"=w394) -> ()  [unwired: 2 in, 2 out]
                }
              }
              "Calculated image plane" <- w386
              "Displayed Hologram" <- w392
            }
          }
        }
        frame True {
        }
      }
      n117 = case shown="True" w273 {
        tunnel: "#images" -> [_ w314]
        tunnel: w288 -> [_ w313]
        tunnel: w287 -> [_ w312]
        tunnel: w286 -> [_ w311]
        tunnel: w285 -> [_ w310]
        tunnel: w278 -> [_ w309]
        tunnel: w284 -> [w298 w306]
        tunnel: [w298 w306] -> w283
        tunnel: w282 -> [_ w305]
        tunnel: w281 -> [_ w304]
        tunnel: w280 -> [_ w303]
        tunnel: w279 -> [_ w302]
        tunnel: w272 -> [_ w301]
        frame False {
        }
        frame True {
          n118 = Wait (ms)(milliseconds to wait=u32 100) -> (millisecond timer value=w300:u32)
          n119 = call <vilib>:"Acquire Semaphore.vi"("semaphore"=w309) -> ("semaphore out"=w308:T11)  [unwired: 4 in, 2 out]
          n120 = for {
            N: w314 -> [_]
            tunnel: w313 -> [w328]
            tunnel: w312 -> [w327]
            tunnel: w311 -> [w326]
            tunnel: w310 -> [w325]
            tunnel: w308 -> [w324]
            tunnel: [w323] -> w307
            tunnel: w305 -> [w321]
            tunnel: w304 -> [w320]
            tunnel: w303 -> [w318]
            tunnel: w302 -> [w317]
            tunnel: w301 -> [w315]
            tunnel: w300 -> [_]
            i -> [w319]
            n121 = Build Array(w321, w320) -> (w316:sgl[][])
            n122 = case shown="True" w318 {
              tunnel: w326 -> [w345 w357]
              tunnel: w328 -> [w344 w356]
              tunnel: [w344 w355] -> _
              tunnel: [w343 w354] -> _
              tunnel: [w345 w353] -> w322
              tunnel: [w346 w352] -> _
              tunnel: w327 -> [w346 w351]
              tunnel: w317 -> [_ w350]
              tunnel: w325 -> [w343 w349]
              tunnel: [_ w348] -> _
              tunnel: w324 -> [w341 w347]
              tunnel: [w341 w347] -> w323
              frame False {
                n123 = Wait (ms)(milliseconds to wait=u32 100) -> ()  [unwired: 1 out]
              }
              frame True {
                n124 = case shown="False" w350 {
                  tunnel: w357 -> [w365 w373]
                  tunnel: [w363 w372] -> w355
                  tunnel: [w362 w371] -> w354
                  tunnel: w356 -> [w363 w370]
                  tunnel: [w364 w369] -> w353
                  tunnel: [w359 w368] -> w348
                  tunnel: [w361 w367] -> w352
                  tunnel: w351 -> [w360 w367]
                  tunnel: w349 -> [w358 w366]
                  frame False {
                    n125 = call <vilib>:"IMAQdx Grab.vi"("error in"=w358, "Image In"=w365, "Session In"=w360) -> ("error out"=w362:errorcluster, "Buffer Number Out"=w359:u32, "Image Out"=w364:T2, "Session Out"=w361:T6)  [unwired: 5 in]
                  }
                  frame True {
                    n126 = call <vilib>:"IMAQ Grab Acquire.vi"("error in (no error)"=w366, "Image In"=w373, "IMAQ Session In"=w370) -> ("error out"=w371:errorcluster, "Acquired Buffer Number"=w368:u32, "Image Out"=w369:T2, "IMAQ Session Out"=w372:refnum<k11>)  [unwired: 1 in, 4 out]
                  }
                }
              }
            }
            n127 = Number To Decimal String(number=w315) -> (decimal integer string=w331:string)  [unwired: 1 in]
            n128 = Number To Decimal String(number=w319) -> (decimal integer string=w333:string)  [unwired: 1 in]
            n129 = Concatenate Strings("Filename", w331, "_" ("string"), w333) -> (w335:string)
            n130 = Concatenate Strings(w335, ".bmp" ("string")) -> (w337:string)
            n131 = Concatenate Strings(w335, "_pos.txt" ("string")) -> (w340:string)
            n132 = Build Path(base path="File Path", name or relative path=w340) -> (appended path=w329:path)
            n133 = Build Path(base path="File Path", name or relative path=w337) -> (appended path=w330:path)
            "appended path" <- w330
            n134 = call-poly <vilib>:"Write To Spreadsheet File.vi"("2D data"=w316, "file path (dialog if empty)"=w329) -> ()  [unwired: 6 in, 1 out]
            n135 = call-poly "IMAQ Write File 2"("File Path"=w330, "Image"=w322) -> ()  [unwired: 8 in, 2 out]
          }
          n136 = call <vilib>:"Release Semaphore.vi"("semaphore"=w307) -> ()  [unwired: 5 in, 2 out]
        }
      }
      "Step number" <- w272
    }
    n137 = local read "Stop program"() -> (w269:bool)
  }
  n138 = call-poly <vilib>:"Close Input Device.vi"("error in (no error)"=w28, "device ID"=w30) -> ()  [unwired: 9 out]
  n139 = for {
    N: 25 -> [_]
    tunnel: [w401] -> w52 mode=indexing
    i -> [w397]
    w399 = T12 1 items=["Grayscale (U8)", "Grayscale (I16)", "Grayscale (SGL)", "Complex (CSG)", "RGB (U32)", "HSL (U32)", "RGB (U64)", "Grayscale (U16)"] ("Image Type")
    n140 = Number To Decimal String(number=w397) -> (decimal integer string=w396:string)  [unwired: 1 in]
    n141 = Concatenate Strings("ROI" ("Image Name"), w396) -> (w398:string)
    n142 = call "IMAQ Create"("Image Name"=w398, "Image Type"=w399) -> ("New Image"=w401:T2)  [unwired: 3 in, 1 out]
  }
  n143 = Obtain Queue(name (unnamed)="Measured Pos data", element data type=T5 {"Centroid X"=[], "Centroid Y"=[], "Acquired Buffer Number"=0} ("output cluster 2")) -> (queue out=w50:refnum<queue>)  [unwired: 3 in, 2 out]
  n144 = Obtain Queue(name (unnamed)="Trap cluster", element data type=w17) -> (queue out=w47:refnum<queue>)  [unwired: 3 in, 2 out]
  n145 = while "Image acquisition loop" {
    tunnel: w5 -> [w411]
    tunnel: w7 -> [w427]
    tunnel: w9 -> [w426]
    tunnel: [w425] -> w54
    tunnel: [w407] -> w53
    tunnel: w52 -> [w421]
    tunnel: w50 -> [w413]
    shift-right: ["ROI size"] -> _
    shift-left: _ -> [_]
    tunnel: w47 -> [w412]
    tunnel: [w421] -> w45
    tunnel: [w408] -> w44
    tunnel: [w420] -> w43
    tunnel: w8 -> [w419]
    tunnel: w4 -> [w418]
    tunnel: w18 -> [w417]
    tunnel: w21 -> [w416]
    tunnel: w6 -> [w414]
    tunnel: w2 -> [w402]
    stop <- w424 stop-if-true
    n146 = Flush Queue(queue=w413) -> ()  [unwired: 1 in, 3 out]
    n147 = Flush Queue(queue=w412) -> ()  [unwired: 1 in, 3 out]
    n148 = Preview Queue Element(queue=w417, timeout in ms (-1)=10 ("f")) -> (element=w406:T3)  [unwired: 1 in, 3 out]
    n149 = call <vilib>:"Acquire Semaphore.vi"("semaphore"=w402) -> ("semaphore out"=w404:T11)  [unwired: 4 in, 2 out]
    n150 = case shown="True" w411 {
      tunnel: w427 -> [w432 w444]
      tunnel: w426 -> [w431 w443]
      tunnel: [w431 w442] -> w425
      tunnel: [w430 w441] -> w407
      tunnel: [w432 w440] -> w408
      tunnel: [w433 w439] -> w420
      tunnel: w419 -> [w433 w438]
      tunnel: w418 -> [_ w437]
      tunnel: w414 -> [w430 w436]
      tunnel: [_ w435] -> _
      tunnel: w404 -> [w428 w434]
      tunnel: [w428 w434] -> w403
      frame False {
        n151 = Wait (ms)(milliseconds to wait=u32 100) -> ()  [unwired: 1 out]
      }
      frame True {
        n152 = case shown="True" w437 {
          tunnel: w444 -> [w452 w460]
          tunnel: [w450 w459] -> w442
          tunnel: [w449 w458] -> w441
          tunnel: w443 -> [w450 w457]
          tunnel: [w451 w456] -> w440
          tunnel: [w446 w455] -> w435
          tunnel: [w448 w454] -> w439
          tunnel: w438 -> [w447 w454]
          tunnel: w436 -> [w445 w453]
          frame False {
            n153 = call <vilib>:"IMAQdx Grab.vi"("error in"=w445, "Image In"=w452, "Session In"=w447) -> ("error out"=w449:errorcluster, "Buffer Number Out"=w446:u32, "Image Out"=w451:T2, "Session Out"=w448:T6)  [unwired: 5 in]
          }
          frame True {
            n154 = call <vilib>:"IMAQ Grab Acquire.vi"("error in (no error)"=w453, "Image In"=w460, "IMAQ Session In"=w457) -> ("error out"=w458:errorcluster, "Acquired Buffer Number"=w455:u32, "Image Out"=w456:T2, "IMAQ Session Out"=w459:refnum<k11>)  [unwired: 1 in, 4 out]
          }
        }
      }
    }
    n155 = Get Queue Status(queue=w416, return elements? (F)="Display path") -> (elements=w409:T3[])  [unwired: 1 in, 7 out]
    n156 = call <vilib>:"Release Semaphore.vi"("semaphore"=w403) -> ()  [unwired: 5 in, 2 out]
    n157 = case shown="True" "Show image" {
      tunnel: w408 -> [_ w461]
      frame False {
      }
      frame True {
        "Image" <- w461
      }
    }
    n158 = call "Create trap overlay.vi"("Current trap cluster"=w406, "Image in"=w408, "ROI size"="ROI size", "Switch X/Y"="Switch X/Y", "Path"=w409) -> ()  [unwired: 1 out]
    n159 = local read "Stop program"() -> (w424:bool)
  }
  n160 = call "IMAQ Dispose"("Image"=w44) -> ()  [unwired: 5 in, 1 out]
  n161 = for {
    tunnel: w45 -> [w462] mode=indexing
    n162 = call "IMAQ Dispose"("Image"=w462) -> ()  [unwired: 5 in, 1 out]
  }
  n163 = case shown="True" w5 {
    tunnel: w54 -> [_ w468]
    tunnel: w53 -> [w463 w467]
    tunnel: w43 -> [_ w466]
    tunnel: w4 -> [_ w465]
    tunnel: [w463 w464] -> w35
    frame False {
    }
    frame True {
      n164 = case shown="False" w465 {
        tunnel: w468 -> [_ w474]
        tunnel: w467 -> [w471 w473]
        tunnel: [w470 w472] -> w464
        tunnel: w466 -> [w469 _]
        frame False {
          n165 = call <vilib>:"IMAQdx Close Camera.vi"("error in"=w471, "Session In"=w469) -> ("error out"=w470:errorcluster)  [unwired: 9 in]
        }
        frame True {
          n166 = call <vilib>:"IMAQ Close.vi"("error in (no error)"=w473, "IMAQ Session In"=w474) -> ("error out"=w472:errorcluster)  [unwired: 9 in]
        }
      }
    }
  }
  n167 = call "FreeGPUandSLM.vi"("error in"=w33) -> ("error out"=w32:errorcluster)  [unwired: 1 out]
  "CUDA/SLM error" <- w32
  n168 = Merge Errors(w35, w34) -> (w31:errorcluster)
  "NI Vision error" <- w31
  n169 = flat-sequence {
    tunnel: w32 -> [_]
    tunnel: w31 -> [_]
    frame #0 {
      n170 = local write "Stop program"(FALSE ("Stop program")) -> ()
    }
  }
